vi "Periodic Tasks.vi"(8 "error in":errorcluster) -> ()   [LabVIEW 2015]
doc: "This VI runs in parallel to other tasks. It can contain as many user-defined periodic loops as you need. These can carry out PID or other sorts of timed response."
uses:
  <vilib>/Rock Robotics/SystemInterfaces/spilib/spi_bus.ctl
  <vilib>/Rock Robotics/WPI/Utilities/WPI_GetSetVariantRefNum.vi
  <vilib>/Rock Robotics/Network Tables/NT Write Number.vi
  Robot Global Data.vi
  C:/Users/12ALEXANDER.TIETSORT/Downloads/ADIS16448-RoboRIO-Driver-master (1)/ADIS16448-RoboRIO-Driver-master/LabVIEW/ADI MXP IMU/FRC ADI MXP IMU.lvlib
panel:
  out "Device Found? 3":bool
  in  "stop 2":bool
  out "IMU Angle Delta 2":cluster{"X":dbl, "Y":dbl, "Z":dbl}
  out "RAW IMU Data 2":T1
  out "IMU AHRS 3":cluster{"Pitch":dbl, "Roll":dbl, "Yaw":dbl}
  out "IMU AHRS Delta 2":cluster{"Pitch":dbl, "Roll":dbl, "Yaw":dbl}
  out "Sensor Ready? 3":bool
  in  "AHRS Yaw Axis":enum16{"X", "Y", "Z"}(ring)=enum."Z"
  out "Sensor Ready? 2":bool
  out "IMU AHRS Delta":cluster{"Pitch":dbl, "Roll":dbl, "Yaw":dbl}
  out "IMU AHRS":cluster{"Pitch":dbl, "Roll":dbl, "Yaw":dbl}
  out "RAW IMU Data":T1
  out "IMU Angle Delta":cluster{"X":dbl, "Y":dbl, "Z":dbl}
  in  "Reset Angles? 2":bool
  out "Device Found? 2":bool
  in  "stop":bool
  # "FRC Analog Devices ADIS16448 IMU Example"
  # "FRC ADI MXP Placement"
  # "Raw IMU Output Data"
  # "IMU Deltas"
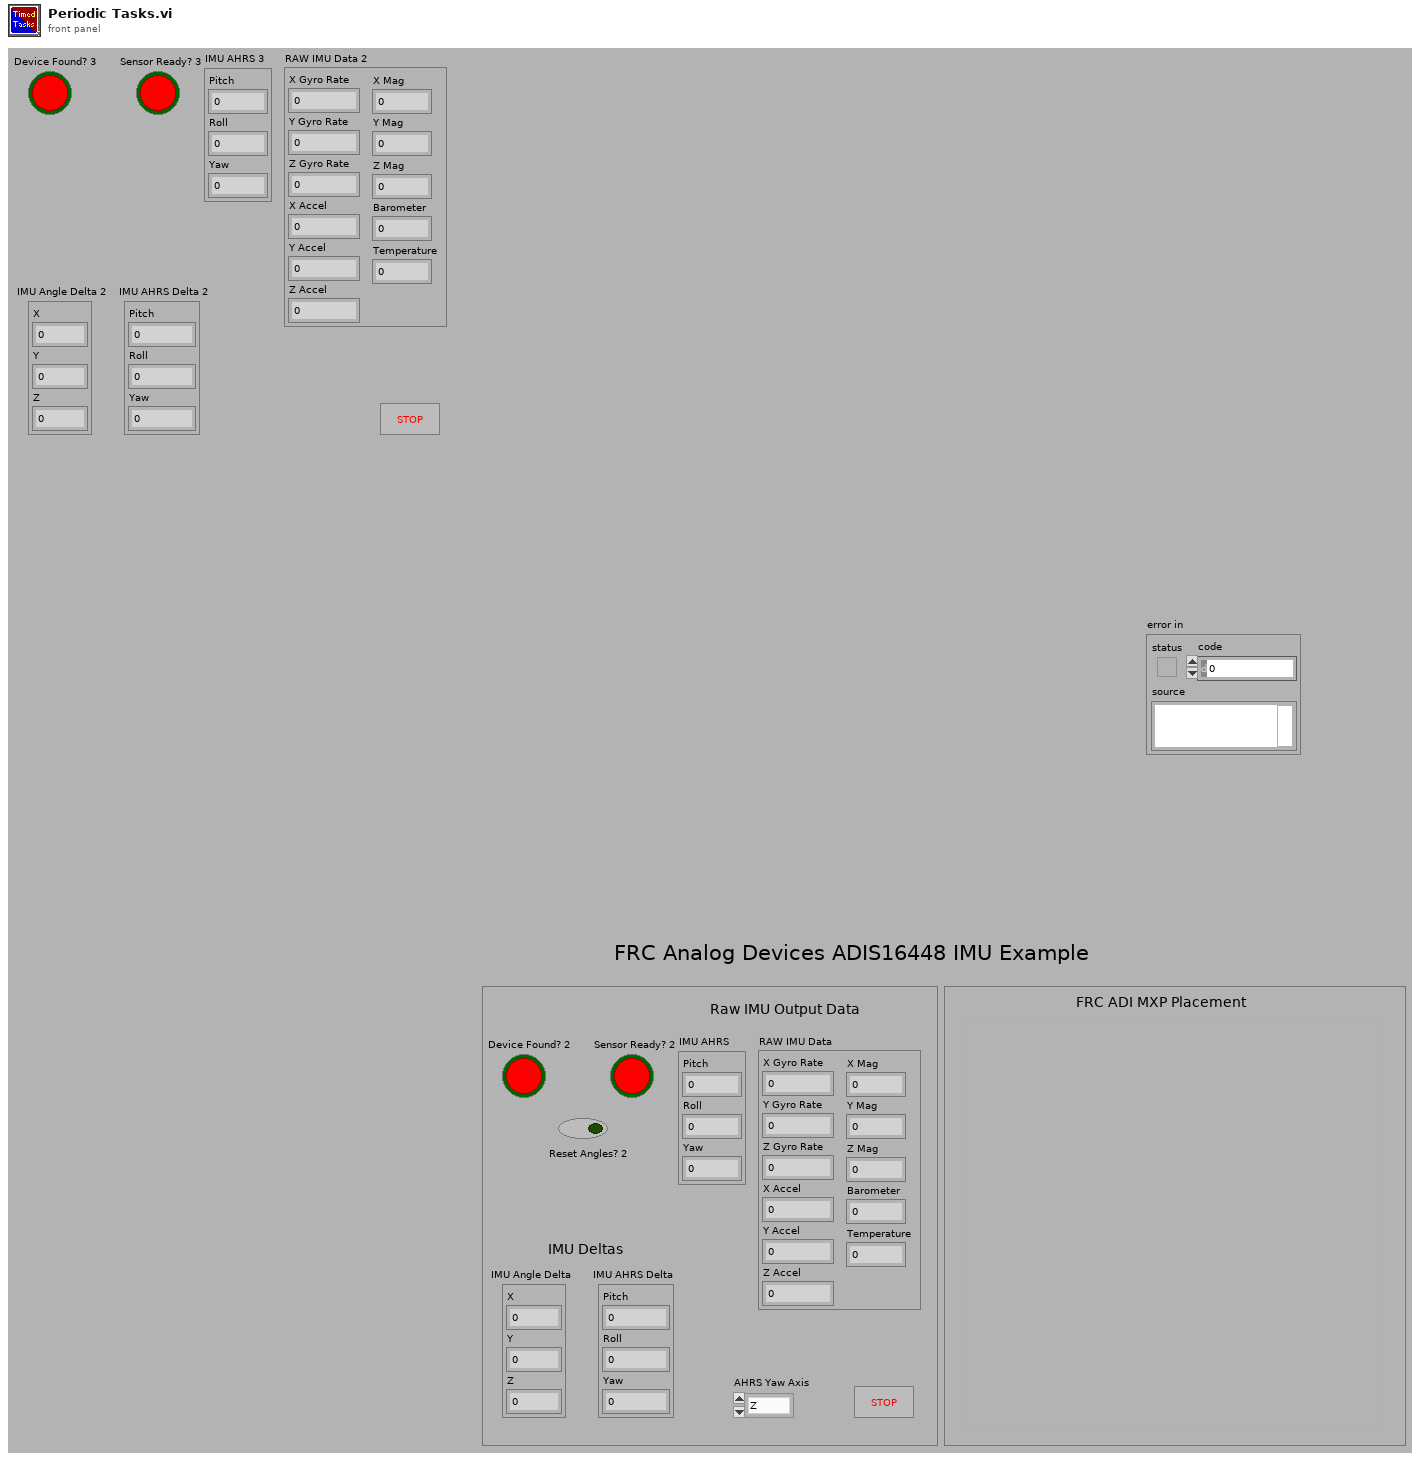
[diagram p1: front panel]
types:
  T1 = cluster{"X Gyro Rate":dbl, "Y Gyro Rate":dbl, "Z Gyro Rate":dbl, "X Accel":dbl, "Y Accel":dbl, "Z Accel":dbl, "X Mag":dbl, "Y Mag":dbl, "Z Mag":dbl, "Barometer":dbl, "Temperature":dbl}
  T2 = typedef "spi_bus.ctl" = enum16{"SPI On-Board, CS0", "SPI On-Board, CS1", "SPI On-Board, CS2", "SPI On-Board, CS3", "SPI MXP", "Invalid"}
  T3 = typedef "WPI_JoystickDevRef.ctl" = cluster{"Device":T4}
  T4 = typedef "WPI_JoystickDeviceEnum.ctl" = enum16{"USB 0", "USB 1", "USB 2", "USB 3", "USB 4", "USB 5"}
  T5 = typedef "WPI_RobotDriveDevRef.ctl" = cluster{"DevStatus":errorcluster, "Motors[]":T6[], "Square Inputs":bool, "Max Output":dbl}
  T6 = typedef "WPI_MotorControlDeviceRef.ctl" = cluster{"DeviceStatus":errorcluster, "Type":T7, "PWM":cluster{"PWM Channel":T8, "DeadBand":T9}, "CAN":cluster{"Device Number":u8, "Control Mode":T10, "Semaphore":T11, "Max Vout":dbl, "TalonSRX Control Mode":T12}, "Invert":bool}
  T7 = typedef "WPI_MotorControlType.ctl" = enum16{"PWM", "CAN", "CANTalonSRX"}
  T8 = typedef "FPGA_DIOPWMChannel.ctl" = enum8{"PWM 0", "PWM 1", "PWM 2", "PWM 3", "PWM 4", "PWM 5", "PWM 6", "PWM 7", "PWM 8", "PWM 9", "PWM MXP 0", "PWM MXP 1", "PWM MXP 2", "PWM MXP 3", "PWM MXP 4", "PWM MXP 5", "PWM MXP 6", "PWM MXP 7", "PWM MXP 8", "PWM MXP 9", "Invalid"}
  T9 = typedef "WPI_PWMDeadband.ctl" = cluster{"Name":string, "maxPositivePwm":i32, "minPositivePwm":i32, "centerPwm":i32, "maxNegativePwm":i32, "minNegativePwm":i32, "angularRange":u16}
  T10 = typedef "WPI_CANJaguar_ControlMode.ctl" = enum8{"Percent VBus", "Current", "Speed", "Position", "Voltage"}
  T11 = typedef "Semaphore RefNum" = refnum<k1>
  T12 = typedef "WPI_CANTalonSRX_APIControlMode.ctl" = enum8{"Percent VBus", "Speed", "Position", "Slave", "Unchanged / Invalid", "Voltage Compensation", "Current", "Motion Profile"}
  T13 = cluster{"JoystickDevRef":T3, "RobotDriveDevRef":T5}
  T14 = typedef "WPI_GyroDevRef.ctl" = cluster{"DevStatus":errorcluster, "Analog Channel":T15, "Offset":dbl, "Gain (VoltsPerDegree/Second)":dbl, "Gyro Type":enum16{"Analog", "XRS450"}, "Handle":i32, "SPI Bus":T2, "Device Found":bool, "Sample Rate":dbl, "Calibrate On Open":bool}
  T15 = typedef "FPGA_AIChannel.ctl" = enum8{"AI 0", "AI 1", "AI 2", "AI 3", "AI MXP 0", "AI MXP 1", "AI MXP 2", "AI MXP 3", "Invalid"}
  T16 = typedef "WPI_AnalogChannelDevRef.ctl" = cluster{"DevStatus":errorcluster, "Analog Channel":T15}
  T17 = typedef "FRC ADI MXP IMU.lvlib/WPI_AnalogDevicesIMUInterruptDevRef.ctl" = cluster{"SimpleGyroDevRef":T18, "InterruptRef":T19}
  T18 = typedef "FRC ADI MXP IMU.lvlib/WPI_AnalogDevicesIMUDevRef.ctl" = cluster{"DevStatus":errorcluster, "Handle":i32, "SPI Bus":T2, "Device Found":bool, "Sample Rate":dbl, "Device Ready":bool, "Yaw Axis":enum16{"X", "Y", "Z"}}
  T19 = typedef "WPI_InterruptRef.ctl" = cluster{"DevStatus":errorcluster, "InterruptIndex":T20}
  T20 = typedef "FPGA_InterruptIndex.ctl" = enum8{"0", "1", "2", "3", "4", "5", "6", "7", "Invalid"}
  T21 = cluster{"X Angle":dbl, "Y Angle":dbl, "Z Angle":dbl}
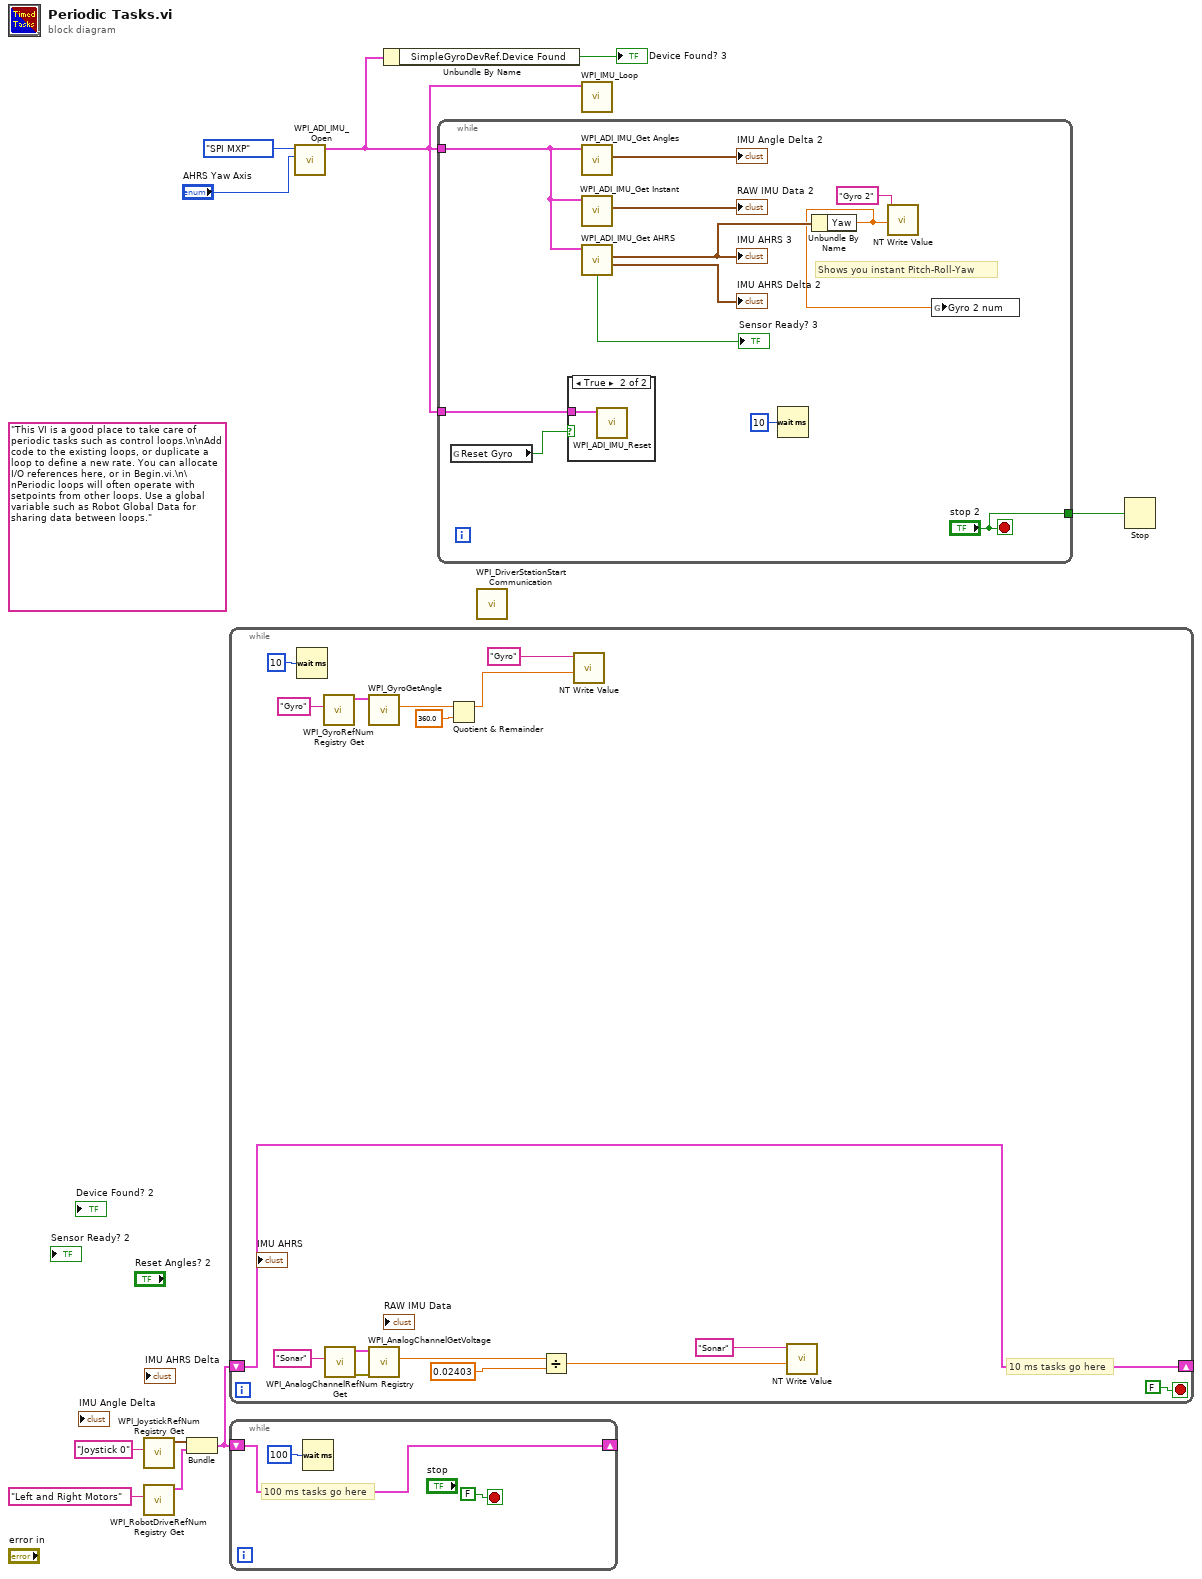
[diagram p0: block diagram]
diagram:
  (unwired) "This VI is a good place to take care of periodic tasks such as control loops.\n\nAdd code to the existing loops, or duplicate a loop to define a new rate. You can allocate I/O references here, or in Begin.vi.\n\nPeriodic loops will often operate with setpoints from other loops. Use a global variable such as Robot Global Data for sharing data between loops."
  n1 = call <vilib>:"WPI_JoystickRefNum Registry Get.vi"("refnum name"="Joystick 0") -> ("JoystickDevRef"=w8:T3)  [unwired: 1 in, 9 out]
  n2 = call <vilib>:"WPI_RobotDriveRefNum Registry Get.vi"("refnum name"="Left and Right Motors") -> ("RobotDriveDevRef"=w7:T5)  [unwired: 1 in, 9 out]
  n3 = Bundle("JoystickDevRef"=w8, "RobotDriveDevRef"=w7) -> (w6:T13)  [unwired: 1 out]
  n4 = while {
    shift-right: [w24] -> _
    shift-left: w6 -> [w24]
    stop <- FALSE stop-if-true
    # "10 ms tasks go here"
    n5 = Wait (ms)(milliseconds to wait=u32 10) -> ()  [unwired: 1 out]
    n6 = call <vilib>:"WPI_GyroRefNum Registry Get.vi"("refnum name"="Gyro") -> ("GyroDevRef"=w13:T14)  [unwired: 9 in, 1 out]
    n7 = call <vilib>:"WPI_AnalogChannelRefNum Registry Get.vi"("refnum name"="Sonar") -> ("error out"=w21:errorcluster, "AIDeviceRef"=w20:T16)  [unwired: 9 in]
    n8 = call <vilib>:"WPI_GyroGetAngle.vi"("GyroDevRef"=w13) -> ("Angle"=w16:dbl)  [unwired: 1 in, 9 out]
    n9 = call <vilib>:"WPI_AnalogChannelGetVoltage.vi"("error in (no error)"=w21, "AIDeviceRef"=w20) -> ("Voltage"=w19:dbl)  [unwired: 7 in, 2 out]
    n10 = Quotient & Remainder(x=w16, y=360.0) -> (x-y*floor(x/y)=w12:dbl)  [unwired: 1 out]
    n11 = Divide(x=w19, y=0.02403) -> (x/y=w17:dbl)
    n12 = call-poly <vilib>:"NT Write Value.vi"("Numeric"=w12, "Name"="Gyro") -> ()  [unwired: 9 in, 1 out]
    n13 = call-poly <vilib>:"NT Write Value.vi"("Numeric"=w17, "Name"="Sonar") -> ()  [unwired: 9 in, 1 out]
  }
  n14 = while {
    shift-right: [w27] -> _
    shift-left: w6 -> [w27]
    stop <- FALSE stop-if-true
    # "100 ms tasks go here"
    n15 = Wait (ms)(milliseconds to wait=u32 100) -> ()  [unwired: 1 out]
  }
  n16 = call "WPI_ADI_IMU_Open.vi"("Yaw Axis"="AHRS Yaw Axis", "SPI Chip Select"=spi_bus."SPI MXP") -> ("ADI IMU Interrupt DevRef"=w2:T17)  [unwired: 8 in, 1 out]
  n17 = Unbundle By Name(w2) -> ("SimpleGyroDevRef.Device Found"=→"Device Found? 3":bool)
  n18 = while {
    tunnel: w2 -> [w35]
    tunnel: ["stop 2"] -> w4
    tunnel: w2 -> [w40]
    stop <- "stop 2" stop-if-true
    # "Shows you instant Pitch-Roll-Yaw"
    n19 = global read "Robot Global Data.vi" "Reset Gyro"() -> (w30:bool)
    n20 = case shown="True" w30 {
      tunnel: w40 -> [_ w42]
      frame False {
      }
      frame True {
        n21 = call "WPI_ADI_IMU_Reset.vi"("ADI IMU Interrupt DevRef"=w42) -> ()  [unwired: 9 in, 2 out]
      }
    }
    n22 = call "WPI_ADI_IMU_Get Angles.vi"("ADI IMU Interrupt DevRef"=w35) -> ("IMU Angles"=→"IMU Angle Delta 2":T21)  [unwired: 7 in, 3 out]
    n23 = call "WPI_ADI_IMU_Get Instant.vi"("ADI IMU Interrupt DevRef"=w35) -> ("IMU Data"=→"RAW IMU Data 2":T1)  [unwired: 7 in, 3 out]
    n24 = call "WPI_ADI_IMU_Get AHRS.vi"("ADI IMU Interrupt DevRef"=w35) -> ("IMU AHRS DELTA"=→"IMU AHRS Delta 2":cluster{"Pitch":dbl, "Roll":dbl, "Yaw":dbl}, "IMU AHRS"=w33:cluster{"Pitch":dbl, "Roll":dbl, "Yaw":dbl}, "Sensor Ready Out"=→"Sensor Ready? 3":bool)  [unwired: 6 in, 2 out]
    "IMU AHRS 3" <- w33
    n25 = Wait (ms)(milliseconds to wait=u32 10) -> ()  [unwired: 1 out]
    n26 = Unbundle By Name(w33) -> ("Yaw"=w31:dbl)
    n27 = call-poly <vilib>:"NT Write Value.vi"("Numeric"=w31, "Name"="Gyro 2") -> ()  [unwired: 9 in, 1 out]
    n28 = global write "Robot Global Data.vi" "Gyro 2 num"(w31) -> ()
  }
  n29 = call <vilib>:"WPI_DriverStationStart Communication.vi"() -> ()  [unwired: 12 in]
  n30 = call "WPI_IMU_Loop.vi"("ADI IMU Interrupt DevRef"=w2) -> ()  [unwired: 10 in, 1 out]
  n31 = Stop(stop? (T)=w4) -> ()
